vi "FlexMag - 24-03-2023.vi"() -> ()   [LabVIEW 2018] (continued)
                                n15152 = local read "ch4 shutdown alg"() -> (w19559:bool)
                                n15153 = local read "ch4_pcgv_gui"() -> (w19555:bool)
                                n15154 = local read "abort ch4"() -> (w19557:bool)
                                n15155 = Wait Until Next ms Multiple(millisecond multiple=u32 200) -> ()  [unwired: 1 out]
                                n15156 = Not(x=w19559) -> (.not. x?=w19558:bool)
                                n15157 = Compound Arithmetic op=OR(w19555, w19557, w19558) -> (w19556:bool)
                                }
                              }
                            }
                          }
                        }
                      }
                      frame True {
                      }
                    }
                  }
                }
              }
              frame #16 {
                n15158 = local read "ch4 shutdown alg"() -> (w19565:bool)
                n15159 = case shown="True" w19565 {
                  frame False {
                  }
                  frame True {
                    n15160 = local read "abort ch4"() -> (w19566:bool)
                    n15161 = case shown="False" w19566 {
                      frame False {
                        n15162 = local read "ch4 vent?"() -> (w19567:bool)
                        n15163 = case shown="True" w19567 {
                          frame False {
                            n15164 = local write "ch4 sd pcgv close led"(TRUE ("ch1 sd cc close led")) -> ()
                            n15165 = Wait (ms)(milliseconds to wait=u32 1000) -> ()  [unwired: 1 out]
                          }
                          frame True {
                            n15166 = local write "ch4 sd pcgv open led"(TRUE ("ch1 sd cc close led")) -> ()
                            n15167 = Wait (ms)(milliseconds to wait=u32 1000) -> ()  [unwired: 1 out]
                          }
                        }
                      }
                      frame True {
                      }
                    }
                  }
                }
              }
              frame #17 {
                n15168 = local read "ch4 shutdown alg"() -> (w19572:bool)
                n15169 = case shown="True" w19572 {
                  frame False {
                  }
                  frame True {
                    n15170 = local read "abort ch4"() -> (w19573:bool)
                    n15171 = case shown="False" w19573 {
                      frame False {
                        n15172 = local read "ch4 vent?"() -> (w19574:bool)
                        n15173 = case shown="True" w19574 {
                          frame False {
                            n15174 = while {
                              i -> [w19581]
                              stop <- w19577 stop-if-true
                              n15175 = Greater Or Equal?(x=w19581, y=200) -> (x >= y?=w19583:bool)
                              n15176 = case shown="True" w19583 {
                                frame False {
                                }
                                frame True {
                                n15177 = local write "ch1 shutdown error"(TRUE ("ch1 pumpdown error")) -> ()
                                n15178 = local write "Warning Message"("CH1 ShutDown process  is canceled !\nCH1 Trns BP Left couldn't be closed" ("Warning Message")) -> ()
                                }
                              }
                              n15179 = local read "CH1_Trns_BP_Left_DI"() -> (w19576:bool)
                              n15180 = case shown="True" w19576 {
                                tunnel: [TRUE FALSE] -> w19575
                                frame False {
                                }
                                frame True {
                                n15181 = Wait Until Next ms Multiple(millisecond multiple=u32 200) -> ()  [unwired: 1 out]
                                n15182 = local write "CH1_Trns_BP_Left_DO"(FALSE ("CH1_WFC_DO")) -> ()
                                }
                              }
                              n15183 = local read "abort ch1"() -> (w19578:bool)
                              n15184 = local read "ch1 shutdown alg"() -> (w19580:bool)
                              n15185 = Not(x=w19580) -> (.not. x?=w19579:bool)
                              n15186 = Compound Arithmetic op=OR(w19575, w19578, w19579) -> (w19577:bool)
                            }
                          }
                          frame True {
                            n15187 = local read "ch3_4 vacuum level"() -> (w19590:string)
                            n15188 = Equal?(x=w19590, y="VACUUM") -> (x = y?=w19591:bool)
                            n15189 = case shown="True" w19591 {
                              frame False {
                              }
                              frame True {
                                n15190 = while {
                                i -> [w19599]
                                stop <- w19595 stop-if-true
                                n15191 = Greater Or Equal?(x=w19599, y=100) -> (x >= y?=w19601:bool)
                                n15192 = case shown="True" w19601 {
                                frame False {
                                }
                                frame True {
                                n15193 = local write "ch4 shutdown error"(TRUE ("ch1 pumpdown error")) -> ()
                                n15194 = local write "Warning Message"("CH4 ShutDown process  is canceled !\nCH4 Trns BP Left couldn't be opened" ("Warning Message")) -> ()
                                }
                                }
                                n15195 = local read "CH4_Trns_BP_Right_DI"() -> (w19594:bool)
                                n15196 = case shown="False" w19594 {
                                tunnel: [FALSE TRUE] -> w19593
                                frame False {
                                n15197 = Wait Until Next ms Multiple(millisecond multiple=u32 200) -> ()  [unwired: 1 out]
                                n15198 = local write "CH4_Trns_BP_Right_DO"(TRUE ("CH1_WFC_DO")) -> ()
                                }
                                frame True {
                                }
                                }
                                n15199 = local read "ch4 shutdown alg"() -> (w19598:bool)
                                n15200 = local read "abort ch4"() -> (w19596:bool)
                                n15201 = Not(x=w19598) -> (.not. x?=w19597:bool)
                                n15202 = Compound Arithmetic op=OR(w19593, w19596, w19597) -> (w19595:bool)
                                }
                              }
                            }
                          }
                        }
                      }
                      frame True {
                      }
                    }
                  }
                }
              }
              frame #18 {
                n15203 = local read "ch4 shutdown alg"() -> (w19608:bool)
                n15204 = case shown="True" w19608 {
                  frame False {
                  }
                  frame True {
                    n15205 = local read "abort ch4"() -> (w19609:bool)
                    n15206 = case shown="False" w19609 {
                      frame False {
                        n15207 = local read "ch4 vent?"() -> (w19610:bool)
                        n15208 = case shown="False" w19610 {
                          frame False {
                            n15209 = local write "ch4 sd trns bp right close led"(TRUE ("ch1 sd cc close led")) -> ()
                            n15210 = Wait (ms)(milliseconds to wait=u32 1000) -> ()  [unwired: 1 out]
                          }
                          frame True {
                            n15211 = local write "ch4 sd trns bp right open led"(TRUE ("ch1 sd cc close led")) -> ()
                            n15212 = Wait (ms)(milliseconds to wait=u32 1000) -> ()  [unwired: 1 out]
                          }
                        }
                      }
                      frame True {
                      }
                    }
                  }
                }
              }
              frame #19 {
                n15213 = local read "ch4 shutdown alg"() -> (w19615:bool)
                n15214 = case shown="True" w19615 {
                  frame False {
                  }
                  frame True {
                    n15215 = local read "abort ch4"() -> (w19616:bool)
                    n15216 = case shown="False" w19616 {
                      frame False {
                        n15217 = local read "ch4 vent?"() -> (w19617:bool)
                        n15218 = case shown="True" w19617 {
                          frame False {
                          }
                          frame True {
                            n15219 = while {
                              i -> [w19620]
                              stop <- w19623 stop-if-true
                              n15220 = Greater?(x=w19620, y=100) -> (0:w19619:bool)
                              n15221 = case shown="True" w19619 {
                                frame False {
                                }
                                frame True {
                                n15222 = local write "Warning Message"("CH4 ShutDown process  is canceled !\nCH4 CH VBV couldn't be opened" ("Warning Message")) -> ()
                                n15223 = local write "ch4 shutdown error"(TRUE ("ch1 pumpdown error")) -> ()
                                }
                              }
                              n15224 = local read "CH4_CH_VBV_DI"() -> (w19618:bool)
                              n15225 = case shown="False" w19618 {
                                tunnel: [FALSE TRUE] -> w19622
                                frame False {
                                n15226 = Wait Until Next ms Multiple(millisecond multiple=u32 200) -> ()  [unwired: 1 out]
                                n15227 = local write "CH4_CH_VBV_DO"(TRUE ("CH1_WFC_DO")) -> ()
                                }
                                frame True {
                                }
                              }
                              n15228 = local read "abort ch4"() -> (w19626:bool)
                              n15229 = local read "ch4 shutdown alg"() -> (w19624:bool)
                              n15230 = Not(x=w19624) -> (.not. x?=w19625:bool)
                              n15231 = Compound Arithmetic op=OR(w19622, w19626, w19625) -> (w19623:bool)
                            }
                          }
                        }
                      }
                      frame True {
                      }
                    }
                  }
                }
              }
              frame #20 {
                n15232 = local read "ch4 shutdown alg"() -> (w19633:bool)
                n15233 = case shown="True" w19633 {
                  frame False {
                  }
                  frame True {
                    n15234 = local read "abort ch4"() -> (w19634:bool)
                    n15235 = case shown="False" w19634 {
                      frame False {
                        n15236 = local read "ch4 vent?"() -> (w19635:bool)
                        n15237 = case shown="True" w19635 {
                          frame False {
                          }
                          frame True {
                            n15238 = local write "ch4 sd ch vbv open led"(TRUE ("ch1 sd cc close led")) -> ()
                            n15239 = Wait (ms)(milliseconds to wait=u32 1000) -> ()  [unwired: 1 out]
                          }
                        }
                      }
                      frame True {
                      }
                    }
                  }
                }
              }
              frame #21 {
                n15240 = local read "ch4 shutdown alg"() -> (w19638:bool)
                n15241 = case shown="True" w19638 {
                  frame False {
                  }
                  frame True {
                    n15242 = local read "abort ch4"() -> (w19639:bool)
                    n15243 = case shown="False" w19639 {
                      frame False {
                        n15244 = local read "ch4 vent?"() -> (w19640:bool)
                        n15245 = case shown="True" w19640 {
                          frame False {
                            n15246 = while {
                              i -> [w19647]
                              stop <- w19643 stop-if-true
                              # "10min"
                              n15247 = Greater Or Equal?(x=w19647, y=3000) -> (x >= y?=w19649:bool)
                              n15248 = case shown="True" w19649 {
                                frame False {
                                }
                                frame True {
                                n15249 = local write "ch4 shutdown error"(TRUE ("ch1 pumpdown error")) -> ()
                                n15250 = local write "Warning Message"("CH4 ShutDown process  is canceled !\nCH4 PL ATM switch  couldn't be opened" ("Warning Message")) -> ()
                                }
                              }
                              n15251 = local read "CH4_PL_ATM_DI"() -> (w19641:bool)
                              n15252 = local read "abort ch4"() -> (w19644:bool)
                              n15253 = local read "ch4 shutdown alg"() -> (w19646:bool)
                              n15254 = case shown="False" w19641 {
                                tunnel: [FALSE TRUE] -> w19642
                                frame False {
                                n15255 = Wait Until Next ms Multiple(millisecond multiple=u32 200) -> ()  [unwired: 1 out]
                                }
                                frame True {
                                }
                              }
                              n15256 = Not(x=w19646) -> (.not. x?=w19645:bool)
                              n15257 = Compound Arithmetic op=OR(w19642, w19644, w19645) -> (w19643:bool)
                            }
                          }
                          frame True {
                            n15258 = while {
                              i -> [w19663]
                              stop <- w19659 stop-if-true
                              # "10min"
                              n15259 = Greater Or Equal?(x=w19663, y=3000) -> (x >= y?=w19665:bool)
                              n15260 = case shown="True" w19665 {
                                frame False {
                                }
                                frame True {
                                n15261 = local write "ch4 shutdown error"(TRUE ("ch1 pumpdown error")) -> ()
                                n15262 = local write "Warning Message"("CH4 ShutDown process  is canceled !\nCH4 ATM switches  couldn't be opened" ("Warning Message")) -> ()
                                }
                              }
                              n15263 = local read "CH4_CH_ATM_DI"() -> (w19657:bool)
                              n15264 = local read "CH4_PL_ATM_DI"() -> (w19656:bool)
                              n15265 = And(x=w19657, y=w19656) -> (x .and. y?=w19655:bool)
                              n15266 = local read "abort ch4"() -> (w19660:bool)
                              n15267 = local read "ch4 shutdown alg"() -> (w19662:bool)
                              n15268 = case shown="False" w19655 {
                                tunnel: [FALSE TRUE] -> w19658
                                frame False {
                                n15269 = Wait Until Next ms Multiple(millisecond multiple=u32 200) -> ()  [unwired: 1 out]
                                }
                                frame True {
                                }
                              }
                              n15270 = Not(x=w19662) -> (.not. x?=w19661:bool)
                              n15271 = Compound Arithmetic op=OR(w19658, w19660, w19661) -> (w19659:bool)
                            }
                          }
                        }
                      }
                      frame True {
                      }
                    }
                  }
                }
              }
              frame #22 {
                n15272 = local read "ch4 shutdown alg"() -> (w19671:bool)
                n15273 = case shown="True" w19671 {
                  frame False {
                  }
                  frame True {
                    n15274 = local read "abort ch4"() -> (w19672:bool)
                    n15275 = case shown="False" w19672 {
                      frame False {
                        n15276 = local read "ch4 vent?"() -> (w19673:bool)
                        n15277 = case shown="True" w19673 {
                          frame False {
                            n15278 = local write "ch4 sd PL atm on led"(TRUE ("ch1 sd cc close led")) -> ()
                            n15279 = Wait (ms)(milliseconds to wait=u32 1000) -> ()  [unwired: 1 out]
                          }
                          frame True {
                            n15280 = local write "CH4_Trns_BP_Right_DO"(FALSE ("CH4_Trns_BP_Right_DO")) -> ()
                            n15281 = local write "pcgv4 auto close"(TRUE ("pcgv4 auto close")) -> ()
                            n15282 = local write "ch4 sd PL-CH atm on led"(TRUE ("ch1 sd cc close led")) -> ()
                            n15283 = Wait (ms)(milliseconds to wait=u32 500) -> ()  [unwired: 1 out]
                            n15284 = local write "ch3_4 vacuum level"("ATMOSPHERE" ("ch3_4 vacuum level")) -> ()
                          }
                        }
                      }
                      frame True {
                      }
                    }
                  }
                }
              }
              frame #23 {
                n15285 = local read "ch4 shutdown alg"() -> (w19681:bool)
                n15286 = case shown="True" w19681 {
                  frame False {
                  }
                  frame True {
                    n15287 = local read "abort ch4"() -> (w19682:bool)
                    n15288 = case shown="False" w19682 {
                      frame False {
                        n15289 = local read "ch4 vent?"() -> (w19683:bool)
                        n15290 = case shown="True" w19683 {
                          frame False {
                            w19686 = TRUE ("Buzzer DO")
                            n15291 = local write "Buzzer DO"(w19686) -> ()
                            n15292 = local write "ch4 sd completed led"(w19686) -> ()
                            n15293 = Wait (ms)(milliseconds to wait=u32 3000) -> ()  [unwired: 1 out]
                            n15294 = local write "System Status"("CH4 SHUTDOWN PROCESS COMPLETED" ("System Status")) -> ()
                          }
                          frame True {
                            w19687 = TRUE ("Buzzer DO")
                            n15295 = local write "Buzzer DO"(w19687) -> ()
                            n15296 = local write "ch4 sd completed led"(w19687) -> ()
                            n15297 = Wait (ms)(milliseconds to wait=u32 3000) -> ()  [unwired: 1 out]
                            n15298 = local write "System Status"("CH4 VENT PROCESS COMPLETED" ("System Status")) -> ()
                          }
                        }
                      }
                      frame True {
                      }
                    }
                  }
                }
              }
              frame #24 {
                n15299 = local read "ch4 shutdown alg"() -> (w19690:bool)
                n15300 = case shown="True" w19690 {
                  frame False {
                  }
                  frame True {
                    n15301 = local read "abort ch4"() -> (w19691:bool)
                    n15302 = case shown="False" w19691 {
                      frame False {
                        w19693 = FALSE ("Buzzer DO")
                        n15303 = local write "Buzzer DO"(w19693) -> ()
                        n15304 = local write "ch4 shutdown alg"(w19693) -> ()
                        n15305 = local write "Shut Down CH4"(w19693) -> ()
                        n15306 = Wait (ms)(milliseconds to wait=u32 3000) -> ()  [unwired: 1 out]
                        n15307 = local write "System Status"("SEMI-AUTOMATIC MODE " ("System Status")) -> ()
                      }
                      frame True {
                      }
                    }
                  }
                }
              }
            }
          }
          frame True {
          }
        }
      }
    }
  }
  n15308 = while {
    stop <- FALSE stop-if-true
    n15309 = Wait Until Next ms Multiple(millisecond multiple=u32 300) -> ()  [unwired: 1 out]
    n15310 = case shown="True" "ch2 pumpdown alg" {
      frame False {
      }
      frame True {
        n15311 = local read "abort ch2"() -> (w20523:bool)
        n15312 = case shown="False" w20523 {
          frame False {
            n15313 = stacked-sequence {
              frame #0 {
                n15314 = stacked-sequence {
                  frame #0 {
                    n15315 = local write "ch2 pd clear"(TRUE ("ch1 pd clear")) -> ()
                    n15316 = Wait (ms)(milliseconds to wait=u32 100) -> ()  [unwired: 1 out]
                  }
                  frame #1 {
                    n15317 = local write "System Status"("CH2 PUMPDOWN PROCESS IN PROGRESS" ("System Status")) -> ()
                  }
                  frame #2 {
                    n15318 = local read "CH2_DS_DI"() -> (w20527:bool)
                    n15319 = case shown="False" w20527 {
                      frame False {
                        n15320 = stacked-sequence {
                          frame #0 {
                            n15321 = local write "Buzzer DO"(TRUE ("Buzzer DO")) -> ()
                            n15322 = Wait (ms)(milliseconds to wait=u32 100) -> ()  [unwired: 1 out]
                          }
                          frame #1 {
                            n15323 = while {
                              i -> [w20532]
                              stop <- w20535 stop-if-true
                              n15324 = Greater?(x=w20532, y=900) -> (0:w20531:bool)
                              n15325 = case shown="True" w20531 {
                                frame False {
                                }
                                frame True {
                                n15326 = local write "Warning Message"("CH2 PumpDown process  is canceled !\nCH2 Door is open" ("Warning Message")) -> ()
                                n15327 = local write "ch2 pumpdown error"(TRUE ("ch1 pumpdown error")) -> ()
                                }
                              }
                              n15328 = local read "CH2_DS_DI"() -> (w20530:bool)
                              n15329 = case shown="True" w20530 {
                                tunnel: [FALSE TRUE] -> w20534
                                frame False {
                                n15330 = Wait Until Next ms Multiple(millisecond multiple=u32 200) -> ()  [unwired: 1 out]
                                }
                                frame True {
                                n15331 = local write "Buzzer DO"(FALSE ("Buzzer DO")) -> ()
                                }
                              }
                              n15332 = local read "ch2 pumpdown alg"() -> (w20536:bool)
                              n15333 = local read "abort ch2"() -> (w20538:bool)
                              n15334 = Not(x=w20536) -> (.not. x?=w20537:bool)
                              n15335 = Compound Arithmetic op=OR(w20534, w20538, w20537) -> (w20535:bool)
                            }
                          }
                        }
                      }
                      frame True {
                      }
                    }
                  }
                  frame #3 {
                    n15336 = disable-structure shown="Disabled" {
                      frame Disabled {
                        n15337 = while {
                          i -> [w20547]
                          stop <- w20550 stop-if-true
                          n15338 = Greater?(x=w20547, y=900) -> (0:w20546:bool)
                          n15339 = case shown="True" w20546 {
                            frame False {
                            }
                            frame True {
                              n15340 = local write "Warning Message"("CH2 PumpDown process  is canceled !\nCH2 Water Switch couldn't be opened" ("Warning Message")) -> ()
                              n15341 = local write "ch2 pumpdown error"(TRUE ("ch1 pumpdown error")) -> ()
                            }
                          }
                          n15342 = local read "CH2_WFC_DI"() -> (w20545:bool)
                          n15343 = case shown="False" w20545 {
                            tunnel: [FALSE TRUE] -> w20549
                            frame False {
                              n15344 = Wait Until Next ms Multiple(millisecond multiple=u32 200) -> ()  [unwired: 1 out]
                              n15345 = local write "CH2_WFC_DO"(TRUE ("CH1_WFC_DO")) -> ()
                            }
                            frame True {
                            }
                          }
                          n15346 = local read "ch2 pumpdown alg"() -> (w20551:bool)
                          n15347 = local read "abort ch2"() -> (w20553:bool)
                          n15348 = Not(x=w20551) -> (.not. x?=w20552:bool)
                          n15349 = Compound Arithmetic op=OR(w20549, w20553, w20552) -> (w20550:bool)
                        }
                      }
                      frame Enabled {
                      }
                    }
                  }
                }
              }
              frame #1 {
                # "ATM switches close"
                n15350 = local read "ch2 pumpdown alg"() -> (w20560:bool)
                n15351 = case shown="True" w20560 {
                  frame False {
                  }
                  frame True {
                    n15352 = local read "abort ch2"() -> (w20561:bool)
                    n15353 = case shown="False" w20561 {
                      frame False {
                        w20563 = FALSE ("CH1_PL_ATM_DO")
                        n15354 = local write "CH2_PL_ATM_DO"(w20563) -> ()
                        n15355 = local write "CH2_CH_ATM_DO"(w20563) -> ()
                        n15356 = Wait (ms)(milliseconds to wait=u32 3000) -> ()  [unwired: 1 out]
                      }
                      frame True {
                      }
                    }
                  }
                }
              }
              frame #2 {
                n15357 = local read "ch2 pumpdown alg"() -> (w20564:bool)
                n15358 = case shown="True" w20564 {
                  frame False {
                  }
                  frame True {
                    n15359 = local read "abort ch2"() -> (w20565:bool)
                    n15360 = case shown="False" w20565 {
                      frame False {
                        n15361 = local write "ch2 atms close led"(TRUE ("CH1_PL_ATM_DO")) -> ()
                        n15362 = Wait (ms)(milliseconds to wait=u32 1000) -> ()  [unwired: 1 out]
                      }
                      frame True {
                      }
                    }
                  }
                }
              }
              frame #3 {
                # "ch vbv close"
                n15363 = local read "ch2 pumpdown alg"() -> (w20568:bool)
                n15364 = case shown="True" w20568 {
                  frame False {
                  }
                  frame True {
                    n15365 = local read "abort ch2"() -> (w20569:bool)
                    n15366 = case shown="False" w20569 {
                      frame False {
                        n15367 = while {
                          i -> [w20572]
                          stop <- w20575 stop-if-true
                          n15368 = Greater Or Equal?(x=w20572, y=100) -> (x >= y?=w20573:bool)
                          n15369 = case shown="True" w20573 {
                            frame False {
                            }
                            frame True {
                              n15370 = local write "Warning Message"("CH2 PumpDown process  is canceled !\nCH2 CH VBV couldn't be closed" ("Warning Message")) -> ()
                              n15371 = local write "ch2 pumpdown error"(TRUE ("ch1 pumpdown error")) -> ()
                            }
                          }
                          n15372 = local read "CH2_CH_VBV_DI"() -> (w20570:bool)
                          n15373 = local read "ch2 pumpdown alg"() -> (w20578:bool)
                          n15374 = case shown="True" w20570 {
                            tunnel: [TRUE FALSE] -> w20574
                            frame False {
                            }
                            frame True {
                              n15375 = local write "CH2_CH_VBV_DO"(FALSE ("CH1_CH_VBV_DO")) -> ()
                              n15376 = Wait Until Next ms Multiple(millisecond multiple=u32 200) -> ()  [unwired: 1 out]
                            }
                          }
                          n15377 = local read "abort ch2"() -> (w20576:bool)
                          n15378 = Not(x=w20578) -> (.not. x?=w20577:bool)
                          n15379 = Compound Arithmetic op=OR(w20574, w20576, w20577) -> (w20575:bool)
                        }
                      }
                      frame True {
                      }
                    }
                  }
                }
              }
              frame #4 {
                n15380 = local read "ch2 pumpdown alg"() -> (w20585:bool)
                n15381 = case shown="True" w20585 {
                  frame False {
                  }
                  frame True {
                    n15382 = local read "abort ch2"() -> (w20586:bool)
                    n15383 = case shown="False" w20586 {
                      frame False {
                        n15384 = local write "ch2 ch vbv close led"(TRUE ("ch1 ch vbv close")) -> ()
                        n15385 = Wait (ms)(milliseconds to wait=u32 1000) -> ()  [unwired: 1 out]
                      }
                      frame True {
                      }
                    }
                  }
                }
              }
              frame #5 {
                # "pl vbv close"
                n15386 = local read "ch2 pumpdown alg"() -> (w20589:bool)
                n15387 = case shown="True" w20589 {
                  frame False {
                  }
                  frame True {
                    n15388 = local read "abort ch2"() -> (w20590:bool)
                    n15389 = case shown="False" w20590 {
                      frame False {
                        n15390 = while {
                          i -> [w20593]
                          stop <- w20596 stop-if-true
                          n15391 = Greater Or Equal?(x=w20593, y=100) -> (x >= y?=w20594:bool)
                          n15392 = case shown="True" w20594 {
                            frame False {
                            }
                            frame True {
                              n15393 = local write "Warning Message"("CH2 PumpDown process  is canceled !\nCH2 PL VBV couldn't be closed" ("Warning Message")) -> ()
                              n15394 = local write "ch2 pumpdown error"(TRUE ("ch1 pumpdown error")) -> ()
                            }
                          }
                          n15395 = local read "CH2_PL_VBV_DI"() -> (w20591:bool)
                          n15396 = local read "ch2 pumpdown alg"() -> (w20599:bool)
                          n15397 = case shown="True" w20591 {
                            tunnel: [TRUE FALSE] -> w20595
                            frame False {
                            }
                            frame True {
                              n15398 = Wait Until Next ms Multiple(millisecond multiple=u32 200) -> ()  [unwired: 1 out]
                              n15399 = local write "CH2_PL_VBV_DO"(FALSE ("CH1_CH_VBV_DO")) -> ()
                            }
                          }
                          n15400 = local read "abort ch2"() -> (w20597:bool)
                          n15401 = Not(x=w20599) -> (.not. x?=w20598:bool)
                          n15402 = Compound Arithmetic op=OR(w20595, w20597, w20598) -> (w20596:bool)
                        }
                      }
                      frame True {
                      }
                    }
                  }
                }
              }
              frame #6 {
                n15403 = local read "ch2 pumpdown alg"() -> (w20606:bool)
                n15404 = case shown="True" w20606 {
                  frame False {
                  }
                  frame True {
                    n15405 = local read "abort ch2"() -> (w20607:bool)
                    n15406 = case shown="False" w20607 {
                      frame False {
                        n15407 = local write "ch2 pl vbv close led"(TRUE ("ch1 ch vbv close")) -> ()
                        n15408 = Wait (ms)(milliseconds to wait=u32 1000) -> ()  [unwired: 1 out]
                      }
                      frame True {
                      }
                    }
                  }
                }
              }
              frame #7 {
                n15409 = local read "ch2 pumpdown alg"() -> (w20610:bool)
                n15410 = case shown="True" w20610 {
                  frame False {
                  }
                  frame True {
                    n15411 = local read "abort ch2"() -> (w20611:bool)
                    n15412 = case shown="False" w20611 {
                      frame False {
                        n15413 = local read "ch3 ch pg torr"() -> (w20615:dbl)
                        n15414 = local read "CH2_CH_ATM_DI"() -> (w20613:bool)
                        n15415 = Less?(x=w20615, y=0.5) -> (x < y?=w20612:bool)
                        n15416 = And(x=w20613, y=w20612) -> (x .and. y?=w20614:bool)
                        n15417 = case shown="True" w20614 {
                          frame False {
                            # "ch trns bp left close"
                            n15418 = while {
                              i -> [w20619]
                              stop <- w20622 stop-if-true
                              n15419 = Greater Or Equal?(x=w20619, y=100) -> (x >= y?=w20620:bool)
                              n15420 = case shown="True" w20620 {
                                frame False {
                                }
                                frame True {
                                n15421 = local write "Warning Message"("CH2 PumpDown process  is canceled !\nCH2 TRNS BP Left couldn't be closed" ("Warning Message")) -> ()
                                n15422 = local write "ch2 pumpdown error"(TRUE ("ch1 pumpdown error")) -> ()
                                }
                              }
                              n15423 = local read "CH2_Trns_BP_Left_DI"() -> (w20617:bool)
                              n15424 = local read "ch2 pumpdown alg"() -> (w20625:bool)
                              n15425 = case shown="True" w20617 {
                                tunnel: [TRUE FALSE] -> w20621
                                frame False {
                                }
                                frame True {
                                n15426 = local write "CH2_Trns_BP_Left_DO"(FALSE ("CH1_CH_VBV_DO")) -> ()
                                n15427 = Wait Until Next ms Multiple(millisecond multiple=u32 200) -> ()  [unwired: 1 out]
                                }
                              }
                              n15428 = local read "abort ch2"() -> (w20623:bool)
                              n15429 = Not(x=w20625) -> (.not. x?=w20624:bool)
                              n15430 = Compound Arithmetic op=OR(w20621, w20623, w20624) -> (w20622:bool)
                            }
                          }
                          frame True {
                            # "ch trns bp left open"
                            n15431 = while {
                              i -> [w20634]
                              stop <- w20637 stop-if-true
                              n15432 = Greater Or Equal?(x=w20634, y=100) -> (x >= y?=w20635:bool)
                              n15433 = case shown="True" w20635 {
                                frame False {
                                }
                                frame True {
                                n15434 = local write "Warning Message"("CH2 PumpDown process  is canceled !\nCH2 TRNS BP Left couldn't be opened" ("Warning Message")) -> ()
                                n15435 = local write "ch2 pumpdown error"(TRUE ("ch1 pumpdown error")) -> ()
                                }
                              }
                              n15436 = local read "CH2_Trns_BP_Left_DI"() -> (w20632:bool)
                              n15437 = local read "ch2 pumpdown alg"() -> (w20640:bool)
                              n15438 = case shown="False" w20632 {
                                tunnel: [FALSE TRUE] -> w20636
                                frame False {
                                n15439 = local write "CH2_Trns_BP_Left_DO"(TRUE ("CH1_CH_VBV_DO")) -> ()
                                n15440 = Wait Until Next ms Multiple(millisecond multiple=u32 200) -> ()  [unwired: 1 out]
                                }
                                frame True {
                                }
                              }
                              n15441 = local read "abort ch2"() -> (w20638:bool)
                              n15442 = Not(x=w20640) -> (.not. x?=w20639:bool)
                              n15443 = Compound Arithmetic op=OR(w20636, w20638, w20639) -> (w20637:bool)
                            }
                          }
                        }
                      }
                      frame True {
                      }
                    }
                  }
                }
              }
              frame #8 {
                n15444 = local read "ch2 pumpdown alg"() -> (w20647:bool)
                n15445 = case shown="True" w20647 {
                  frame False {
                  }
                  frame True {
                    n15446 = local read "abort ch2"() -> (w20648:bool)
                    n15447 = case shown="False" w20648 {
                      frame False {
                        n15448 = local read "CH2_Trns_BP_Left_DI"() -> (w20649:bool)
                        n15449 = case shown="False" w20649 {
                          frame False {
                            n15450 = local write "ch2 trns bp left close led"(TRUE ("ch1 ch vbv close")) -> ()
                            n15451 = Wait (ms)(milliseconds to wait=u32 1000) -> ()  [unwired: 1 out]
                          }
                          frame True {
                          }
                        }
                      }
                      frame True {
                      }
                    }
                  }
                }
              }
              frame #9 {
                n15452 = local read "ch2 pumpdown alg"() -> (w20652:bool)
                n15453 = case shown="True" w20652 {
                  frame False {
                  }
                  frame True {
                    n15454 = local read "abort ch2"() -> (w20653:bool)
                    n15455 = case shown="False" w20653 {
                      frame False {
                        n15456 = local read "ch1 ch pg torr"() -> (w20656:dbl)
                        n15457 = local read "CH2_CH_ATM_DI"() -> (w20657:bool)
                        n15458 = Less?(x=w20656, y=0.5) -> (x < y?=w20658:bool)
                        n15459 = And(x=w20657, y=w20658) -> (x .and. y?=w20654:bool)
                        n15460 = case shown="False" w20654 {
                          frame False {
                            # "ch trns bp right close"
                            n15461 = while {
                              i -> [w20661]
                              stop <- w20664 stop-if-true
                              n15462 = Greater Or Equal?(x=w20661, y=100) -> (x >= y?=w20662:bool)
                              n15463 = case shown="True" w20662 {
                                frame False {
                                }
                                frame True {
                                n15464 = local write "Warning Message"("CH2 PumpDown process  is canceled !\nCH2 TRNS BP Right couldn't be closed" ("Warning Message")) -> ()
                                n15465 = local write "ch2 pumpdown error"(TRUE ("ch1 pumpdown error")) -> ()
                                }
                              }
                              n15466 = local read "CH2_Trns_BP_Right_DI"() -> (w20659:bool)
                              n15467 = local read "ch2 pumpdown alg"() -> (w20667:bool)
                              n15468 = case shown="True" w20659 {
                                tunnel: [TRUE FALSE] -> w20663
                                frame False {
                                }
                                frame True {
                                n15469 = local write "CH2_Trns_BP_Right_DO"(FALSE ("CH1_CH_VBV_DO")) -> ()
                                n15470 = Wait Until Next ms Multiple(millisecond multiple=u32 200) -> ()  [unwired: 1 out]
                                }
                              }
                              n15471 = local read "abort ch2"() -> (w20665:bool)
                              n15472 = Not(x=w20667) -> (.not. x?=w20666:bool)
                              n15473 = Compound Arithmetic op=OR(w20663, w20665, w20666) -> (w20664:bool)
                            }
                          }
                          frame True {
                            # "ch trns bp right open"
                            n15474 = while {
                              i -> [w20676]
                              stop <- w20679 stop-if-true
                              n15475 = Greater Or Equal?(x=w20676, y=100) -> (x >= y?=w20677:bool)
                              n15476 = case shown="True" w20677 {
                                frame False {
                                }
                                frame True {
                                n15477 = local write "Warning Message"("CH2 PumpDown process  is canceled !\nCH2 TRNS BP Right couldn't be opened" ("Warning Message")) -> ()
                                n15478 = local write "ch2 pumpdown error"(TRUE ("ch1 pumpdown error")) -> ()
                                }
                              }
                              n15479 = local read "CH2_Trns_BP_Right_DI"() -> (w20674:bool)
                              n15480 = local read "ch2 pumpdown alg"() -> (w20682:bool)
                              n15481 = case shown="False" w20674 {
                                tunnel: [FALSE TRUE] -> w20678
                                frame False {
                                n15482 = local write "CH2_Trns_BP_Right_DO"(TRUE ("CH1_CH_VBV_DO")) -> ()
                                n15483 = Wait Until Next ms Multiple(millisecond multiple=u32 200) -> ()  [unwired: 1 out]
                                }
                                frame True {
                                }
                              }
                              n15484 = local read "abort ch2"() -> (w20680:bool)
                              n15485 = Not(x=w20682) -> (.not. x?=w20681:bool)
                              n15486 = Compound Arithmetic op=OR(w20678, w20680, w20681) -> (w20679:bool)
                            }
                          }
                        }
                      }
                      frame True {
                      }
                    }
                  }
                }
              }
              frame #10 {
                n15487 = local read "ch2 pumpdown alg"() -> (w20689:bool)
                n15488 = case shown="True" w20689 {
                  frame False {
                  }
                  frame True {
                    n15489 = local read "abort ch2"() -> (w20690:bool)
                    n15490 = case shown="False" w20690 {
                      frame False {
                        n15491 = local read "CH2_Trns_BP_Right_DI"() -> (w20691:bool)
                        n15492 = case shown="False" w20691 {
                          frame False {
                            n15493 = local write "ch2 trns bp right close led"(TRUE ("ch1 ch vbv close")) -> ()
                            n15494 = Wait (ms)(milliseconds to wait=u32 1000) -> ()  [unwired: 1 out]
                          }
                          frame True {
                          }
                        }
                      }
                      frame True {
                      }
                    }
                  }
                }
              }
              frame #11 {
                # "ch trns gv 1-2 close"
                n15495 = local read "ch2 pumpdown alg"() -> (w20694:bool)
                n15496 = case shown="True" w20694 {
                  frame False {
                  }
                  frame True {
                    n15497 = local read "abort ch2"() -> (w20695:bool)
                    n15498 = case shown="False" w20695 {
                      frame False {
                        n15499 = while {
                          i -> [w20698]
                          stop <- w20701 stop-if-true
                          n15500 = Greater Or Equal?(x=w20698, y=600) -> (x >= y?=w20699:bool)
                          n15501 = case shown="True" w20699 {
                            frame False {
                            }
                            frame True {
                              n15502 = local write "Warning Message"("CH2 PumpDown process  is canceled !\nCH1-CH2 TRNS GV couldn't be closed" ("Warning Message")) -> ()
                              n15503 = local write "ch2 pumpdown error"(TRUE ("ch1 pumpdown error")) -> ()
                            }
                          }
                          n15504 = local read "CH1_Trns_Gv_Close_DI"() -> (w20696:bool)
                          n15505 = case shown="False" w20696 {
                            tunnel: [FALSE TRUE] -> w20700
                            frame False {
                              n15506 = local write "CH1_Trns_Gv_Open_DO"(FALSE ("CH2_Trns_GV_Open_DO")) -> ()
                              n15507 = local write "CH1_Trns_Gv_Close_DO"(TRUE ("CH1_CH_VBV_DO")) -> ()
                              n15508 = Wait Until Next ms Multiple(millisecond multiple=u32 200) -> ()  [unwired: 1 out]
                            }
                            frame True {
                            }
                          }
                          n15509 = local read "ch2 pumpdown alg"() -> (w20704:bool)
                          n15510 = local read "abort ch2"() -> (w20702:bool)
                          n15511 = Not(x=w20704) -> (.not. x?=w20703:bool)
                          n15512 = Compound Arithmetic op=OR(w20700, w20702, w20703) -> (w20701:bool)
                        }
                      }
                      frame True {
                      }
                    }
                  }
                }
              }
              frame #12 {
                n15513 = local read "ch2 pumpdown alg"() -> (w20712:bool)
                n15514 = case shown="True" w20712 {
                  frame False {
                  }
                  frame True {
                    n15515 = local read "abort ch2"() -> (w20713:bool)
                    n15516 = case shown="False" w20713 {
                      frame False {
                        n15517 = local write "ch1-ch2 trns gv close led"(TRUE ("ch1 ch vbv close")) -> ()
                        n15518 = Wait (ms)(milliseconds to wait=u32 1000) -> ()  [unwired: 1 out]
                      }
                      frame True {
                      }
                    }
                  }
                }
              }
              frame #13 {
                # "ch trns gv 2-3 close"
                n15519 = local read "ch2 pumpdown alg"() -> (w20716:bool)
                n15520 = case shown="True" w20716 {
                  frame False {
                  }
                  frame True {
                    n15521 = local read "abort ch2"() -> (w20717:bool)
                    n15522 = case shown="False" w20717 {
                      frame False {
                        n15523 = while {
                          i -> [w20720]
                          stop <- w20723 stop-if-true
                          n15524 = Greater Or Equal?(x=w20720, y=600) -> (x >= y?=w20721:bool)
                          n15525 = case shown="True" w20721 {
                            frame False {
                            }
                            frame True {
                              n15526 = local write "Warning Message"("CH2 PumpDown process  is canceled !\nCH2-CH3 TRNS GV couldn't be closed" ("Warning Message")) -> ()
                              n15527 = local write "ch2 pumpdown error"(TRUE ("ch1 pumpdown error")) -> ()
                            }
                          }
                          n15528 = local read "CH2_Trns_Gv_Close_DI"() -> (w20718:bool)
                          n15529 = case shown="False" w20718 {
                            tunnel: [FALSE TRUE] -> w20722
                            frame False {
                              w20730 = TRUE ("CH1_CH_VBV_DO")
                              n15530 = Not(x=w20730) -> (.not. x?=w20729:bool)
                              n15531 = local write "CH2_Trns_GV_Open_DO"(w20729) -> ()
                              n15532 = local write "CH2_Trns_GV_Close_DO"(w20730) -> ()
                              n15533 = Wait Until Next ms Multiple(millisecond multiple=u32 200) -> ()  [unwired: 1 out]
                            }
                            frame True {
                            }
                          }
                          n15534 = local read "ch2 pumpdown alg"() -> (w20726:bool)
                          n15535 = local read "abort ch2"() -> (w20724:bool)
                          n15536 = Not(x=w20726) -> (.not. x?=w20725:bool)
                          n15537 = Compound Arithmetic op=OR(w20722, w20724, w20725) -> (w20723:bool)
                        }
                      }
                      frame True {
                      }
                    }
                  }
                }
              }
              frame #14 {
                n15538 = local read "ch2 pumpdown alg"() -> (w20734:bool)
                n15539 = case shown="True" w20734 {
                  frame False {
                  }
                  frame True {
                    n15540 = local read "abort ch2"() -> (w20735:bool)
                    n15541 = case shown="False" w20735 {
                      frame False {
                        n15542 = local write "ch2-ch3 trns gv close led"(TRUE ("ch1 ch vbv close")) -> ()
                        n15543 = Wait (ms)(milliseconds to wait=u32 1000) -> ()  [unwired: 1 out]
                      }
                      frame True {
                      }
                    }
                  }
                }
              }
              frame #15 {
                # "tp bv open\npc gv open"
                n15544 = local read "ch2 pumpdown alg"() -> (w20738:bool)
                n15545 = case shown="True" w20738 {
                  frame False {
                  }
                  frame True {
                    n15546 = local read "abort ch2"() -> (w20739:bool)
                    n15547 = case shown="False" w20739 {
                      frame False {
                        n15548 = local read "CH2_CH_ATM_DI"() -> (w20741:bool)
                        n15549 = local read "CH2_PL_ATM_DI"() -> (w20742:bool)
                        n15550 = And(x=w20741, y=w20742) -> (x .and. y?=w20740:bool)
                        n15551 = case shown="True" w20740 {
                          frame False {
                          }
                          frame True {
                            n15552 = stacked-sequence {
                              frame #0 {
                                # "tp bv open\npc gv open"
                              }
                              frame #1 {
                                n15553 = while {
                                i -> [w20745]
                                stop <- w20748 stop-if-true
                                n15554 = Greater Or Equal?(x=w20745, y=100) -> (x >= y?=w20746:bool)
                                n15555 = case shown="True" w20746 {
                                frame False {
                                }
                                frame True {
                                n15556 = local write "Warning Message"("CH2 PumpDown process  is canceled !\nCH2 TP BV couldn't be opened" ("Warning Message")) -> ()
                                n15557 = local write "ch2 pumpdown error"(TRUE ("ch1 pumpdown error")) -> ()
                                }
                                }
                                n15558 = local read "CH2_TP_BV_DI"() -> (w20743:bool)
                                n15559 = local read "ch2 pumpdown alg"() -> (w20751:bool)
                                n15560 = case shown="False" w20743 {
                                tunnel: [FALSE TRUE] -> w20747
                                frame False {
                                n15561 = Wait Until Next ms Multiple(millisecond multiple=u32 200) -> ()  [unwired: 1 out]
                                n15562 = local write "CH2_TP_BV_DO"(TRUE ("CH1_CH_VBV_DO")) -> ()
                                }
                                frame True {
                                }
                                }
                                n15563 = local read "abort ch2"() -> (w20749:bool)
                                n15564 = Not(x=w20751) -> (.not. x?=w20750:bool)
                                n15565 = Compound Arithmetic op=OR(w20747, w20749, w20750) -> (w20748:bool)
                                }
                              }
                              frame #2 {
                                n15566 = local read "ch2 pumpdown alg"() -> (w20758:bool)
                                n15567 = case shown="True" w20758 {
                                frame False {
                                }
                                frame True {
                                n15568 = local write "ch2 tp bv open led"(TRUE ("ch1 tp bv open led")) -> ()
                                n15569 = Wait (ms)(milliseconds to wait=u32 1000) -> ()  [unwired: 1 out]
                                }
                                }
                              }
                              frame #3 {
                                n15570 = stacked-sequence {
                                frame #0 {
                                n15571 = local read "ch2 pumpdown alg"() -> (w20761:bool)
                                n15572 = case shown="True" w20761 {
                                frame False {
                                }
                                frame True {
                                n15573 = flat-sequence {
                                frame #0 {
                                n15574 = local write "pcgv2 auto open"(TRUE ("pcgv1 auto open")) -> ()
                                }
                                frame #1 {
                                n15575 = Wait (ms)(milliseconds to wait=u32 2000) -> ()  [unwired: 1 out]
                                }
                                frame #2 {
                                n15576 = local write "pcgv2 auto open"(TRUE ("pcgv1 auto open")) -> ()
                                }
                                }
                                }
                                }
                                }
                                frame #1 {
                                n15577 = while {
                                i -> [w20771]